vi "StarlyteWeatherLocationComparison.vi"() -> ()   [LabVIEW 2013]
doc: "# STARLYTE WEATHER LOCATION COMPARISON\n# SUBMITTED FOR 2017 NASA INTERNATIONAL SPACE APPS CHALLENGE\n# PROJECT: STARLYTE\n# AUTHORS: ANDREW DENIO\n# DATE: 5/5/2017"
uses:
  <vilib>/regexp/Match Regular Expression.xnode
panel:
  out "output string 3":string
  out "output string 2":string
  out "output string":string
  in  "stop":bool
  out "Fayetteville":picture
  out "HI-SEAs":picture
  out "element 126":string
  out "element 125":string
  out "element 124":string
  out "element 123":string
  out "element 122":string
  out "element 121":string
  out "element 120":string
  out "element 119":string
  out "element 118":string
  out "element 117":string
  out "element 116":string
  out "element 115":string
  out "element 114":string
  out "element 113":string
  out "element 112":string
  out "element 111":string
  out "element 110":string
  out "element 109":string
  out "element 84":string
  out "element 83":string
  out "element 82":string
  out "element 81":string
  out "element 80":string
  out "element 79":string
  out "element 78":string
  out "element 77":string
  out "element 76":string
  out "element 75":string
  out "element 74":string
  out "element 73":string
  out "element 72":string
  out "element 71":string
  out "element 70":string
  out "element 69":string
  out "element 68":string
  out "element 67":string
  out "element 66":string
  out "element 65":string
  out "element 64":string
  out "element 63":string
  out "element 62":string
  out "element 61":string
  out "element 60":string
  out "element 59":string
  out "element 58":string
  out "element 57":string
  out "element 56":string
  out "element 55":string
  out "element 54":string
  out "element 53":string
  out "element 52":string
  out "element 51":string
  out "element 50":string
  out "element 49":string
  out "element 48":string
  out "element 47":string
  out "element 46":string
  out "element 45":string
  out "element 44":string
  out "element 43":string
  out "element 42":string
  out "element 41":string
  out "element 40":string
  out "element 39":string
  out "element 38":string
  out "element 37":string
  out "element 36":string
  out "element 35":string
  out "element 34":string
  out "element 33":string
  out "element 32":string
  out "element 31":string
  out "element 30":string
  out "element 29":string
  out "element 28":string
  out "element 27":string
  out "element 26":string
  out "element 25":string
  out "element 24":string
  out "element 23":string
  out "element 22":string
  out "element 21":string
  out "element 20":string
  out "element 19":string
  out "element 18":string
  out "element 17":string
  out "element 16":string
  out "element 15":string
  out "element 14":string
  out "element 13":string
  out "element 12":string
  out "element 11":string
  out "element 10":string
  out "element 9":string
  out "element 8":string
  out "element 7":string
  out "element 6":string
  out "element 5":string
  out "element 4":string
  out "element 3":string
  out "element 2":string
  out "element":string
  # "HI-SEAs"
  # "Fayetteville"
  # "Space"
  # "Weather Location Comparison"
  # "Lattitude / Longitude:"
  # "Lattitude / Longitude:"
  # "Lattitude / Longitude:"
  # "Local Time:"
  # "Local Time:"
  # "Local Time:"
  # "Observation Time:"
  # "Observation Time:"
  # "Observation Time:"
  # "Station ID:"
  # "Station ID:"
  # "Station ID:"
  # "Local City:"
  # "Local City:"
  # "Local City:"
  # "Elevation:"
  # "Elevation:"
  # "Elevation:"
  # "Weather Alerts:"
  # "Weather Alerts:"
  # "Weather Alerts:"
  # "Condition:"
  # "Condition:"
  # "Condition:"
  # "Solar Radiation (W/m^2):"
  # "Solar Radiation (W/m^2):"
  # "Solar Radiation (W/m^2):"
  # "Current Temp (F):"
  # "Current Temp (F):"
  # "Current Temp (F):"
  # "Feels Like (F):"
  # "Feels Like (F):"
  # "Feels Like (F):"
  # "Wind Direction:"
  # "Wind Direction:"
  # "Wind Direction:"
  # "Wind Speed (mph):"
  # "Wind Speed (mph):"
  # "Wind Speed (mph):"
  # "Pressure (mb):"
  # "Pressure (mb):"
  # "Pressure (mb):"
  # "Precipitation (in):"
  # "Precipitation (in):"
  # "Precipitation (in):"
  # "Humidity:"
  # "Humidity:"
  # "Humidity:"
  # "Sunrise:"
  # "Sunrise:"
  # "Sunrise:"
  # "Sunset:"
  # "Sunset:"
  # "Sunset:"
  # "Instant Power:"
  # "Instant Power:"
  # "Instant Power:"
  # "Forecast:"
  # "Radar:"
  # "Forecast:"
  # "+1 Day:"
  # "+2 Days:"
  # "+3 Days:"
  # "+1 Day:"
  # "+2 Days:"
  # "+3 Days:"
  # "Condition:"
  # "Condition:"
  # "High Temp (F):"
  # "High Temp (F):"
  # "Low Temp (F):"
  # "Low Temp (F):"
  # "Chance of Rain (%):"
  # "Chance of Rain (%):"
  # "Rain level (in):"
  # "Rain level (in):"
  # "Wind Speed (mph):"
  # "Wind Speed (mph):"
  # "Wind Direction:"
  # "Wind Direction:"
  # "Avg Humidity (%)"
  # "Avg Humidity (%)"
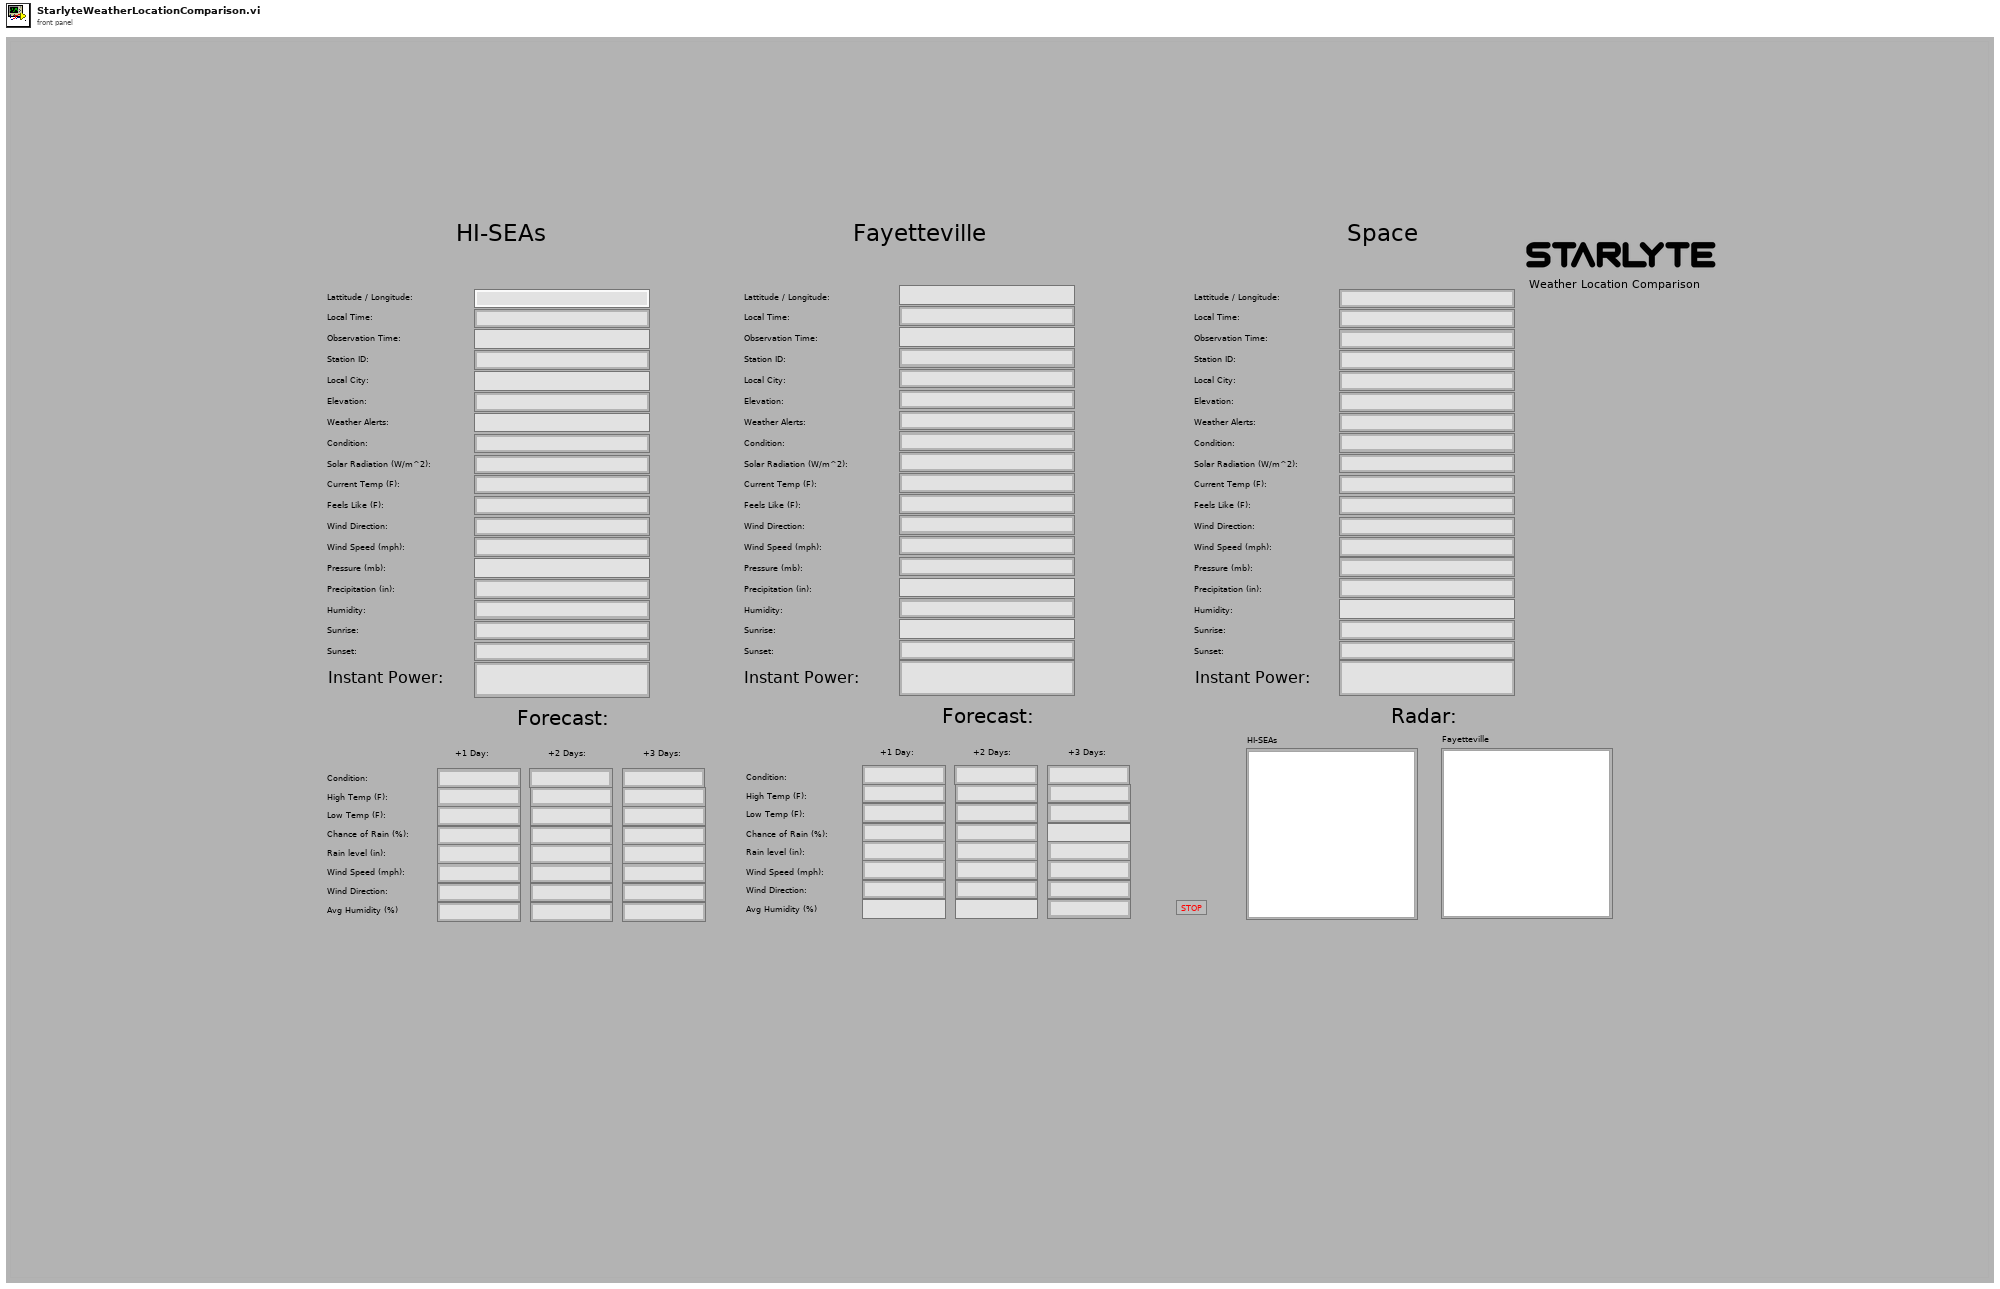
[diagram p1: front panel]
types:
  T1 = typedef "imagedata.ctl" = cluster{"image type":i32, "image depth":i32, "image":u8[], "mask":u8[], "colors":u32[], "Rectangle":cluster{"left":i16, "top":i16, "right":i16, "bottom":i16}}
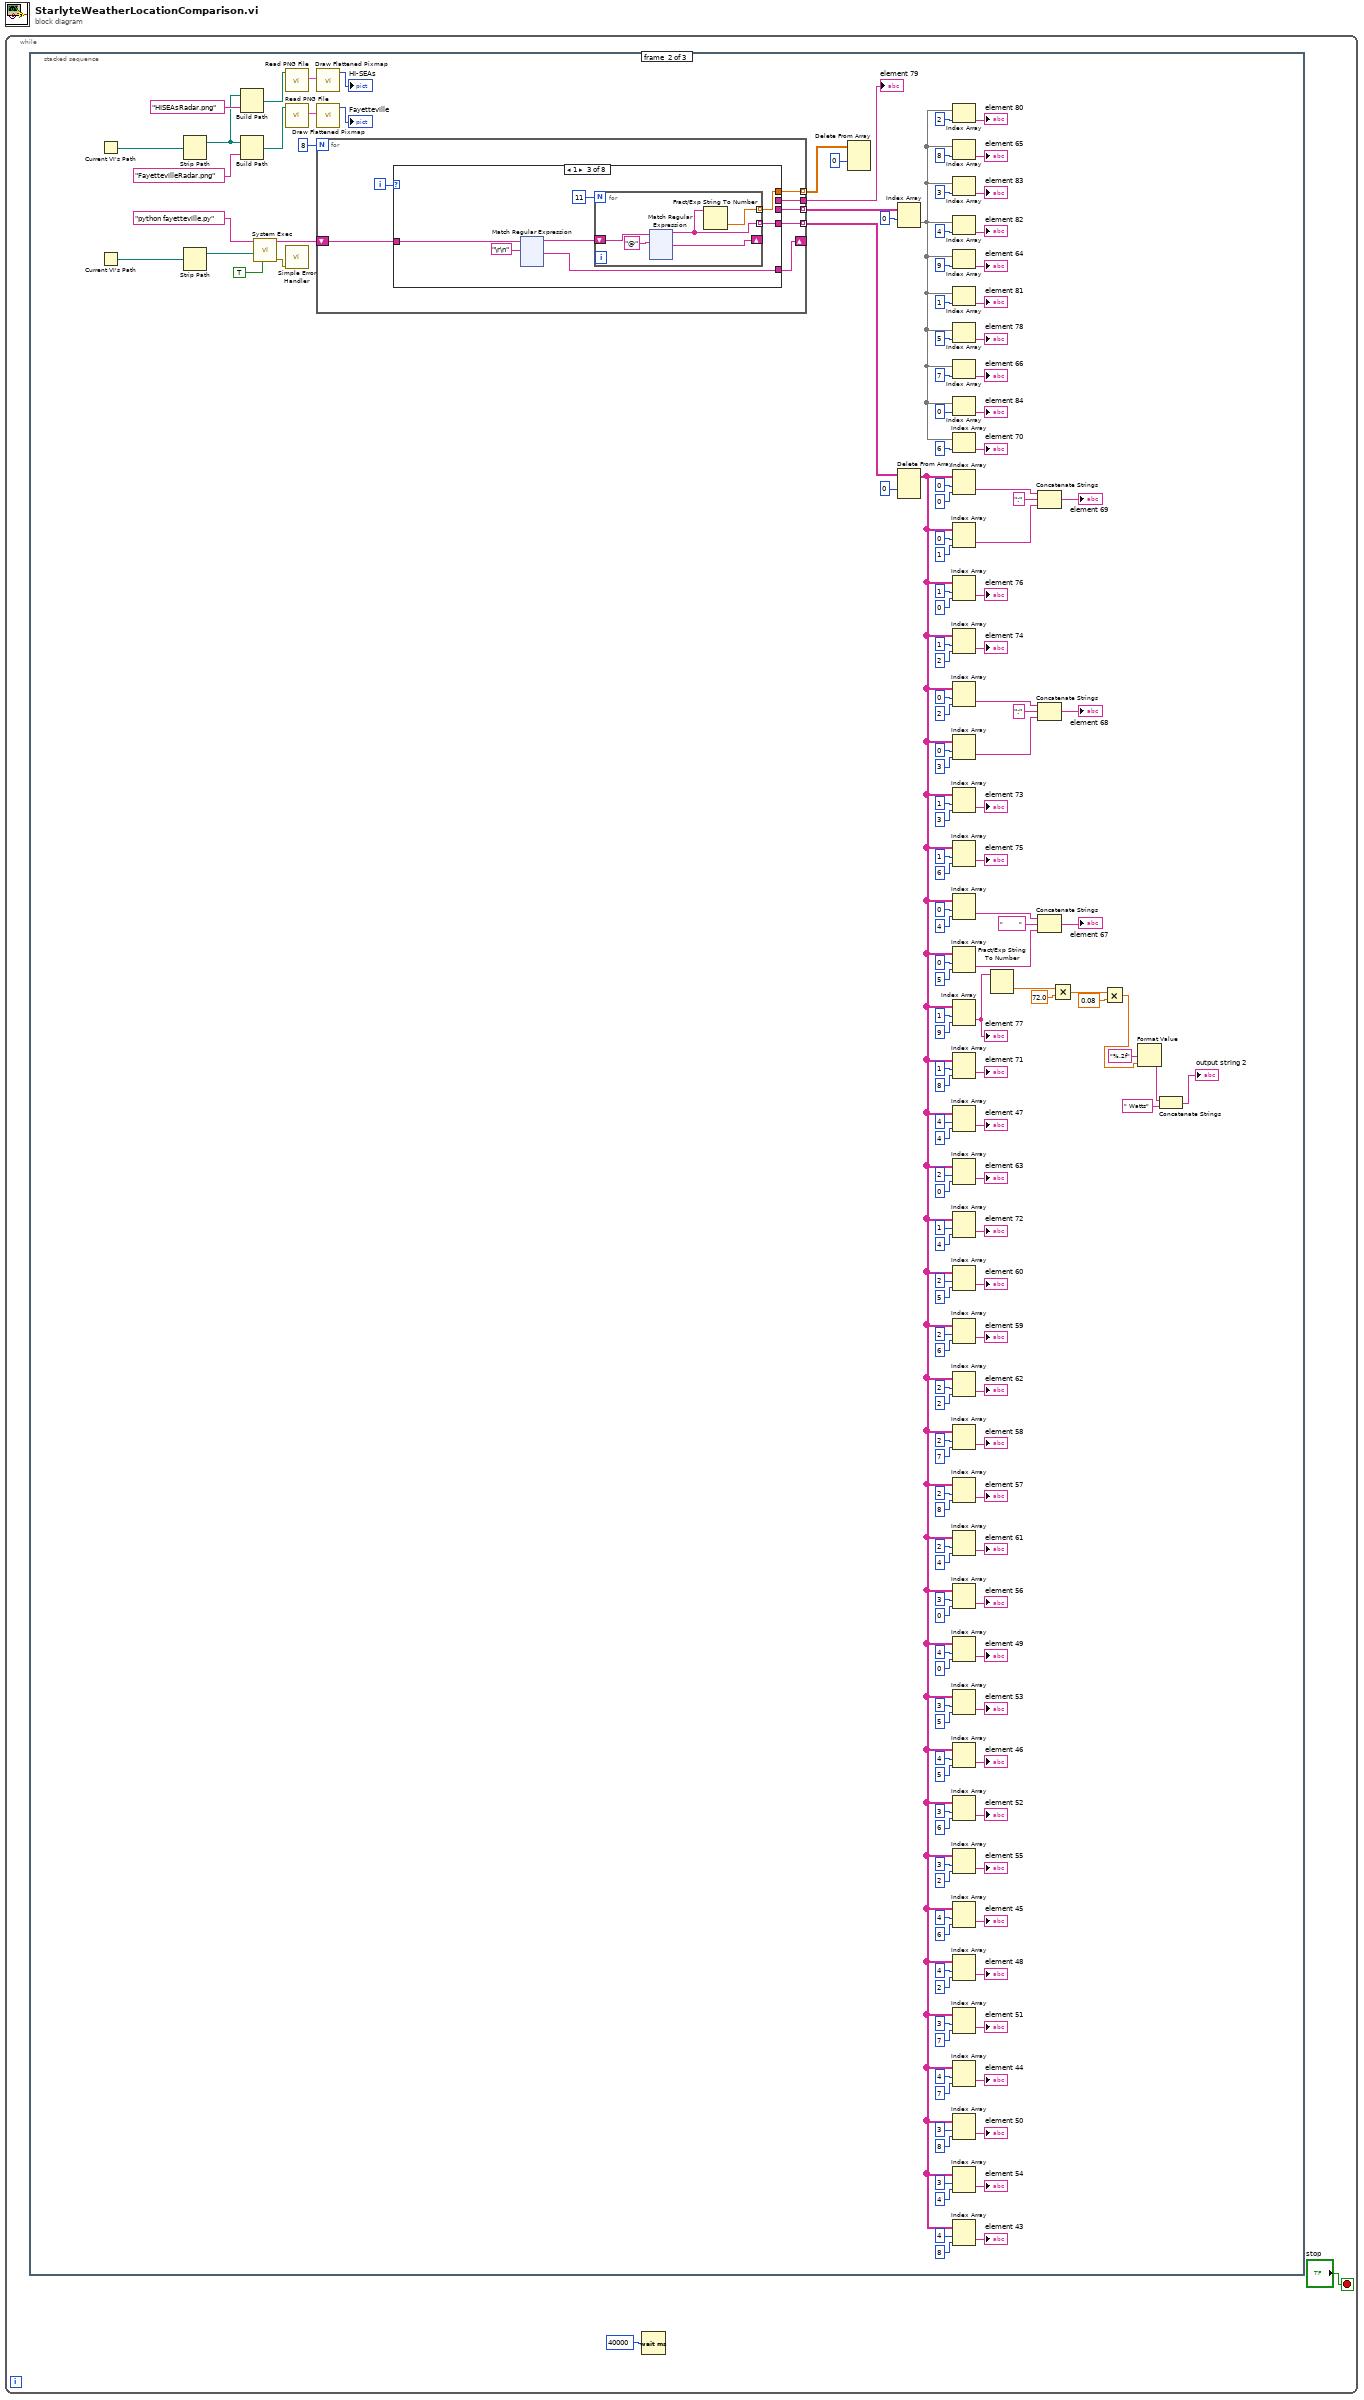
[diagram p0: block diagram]
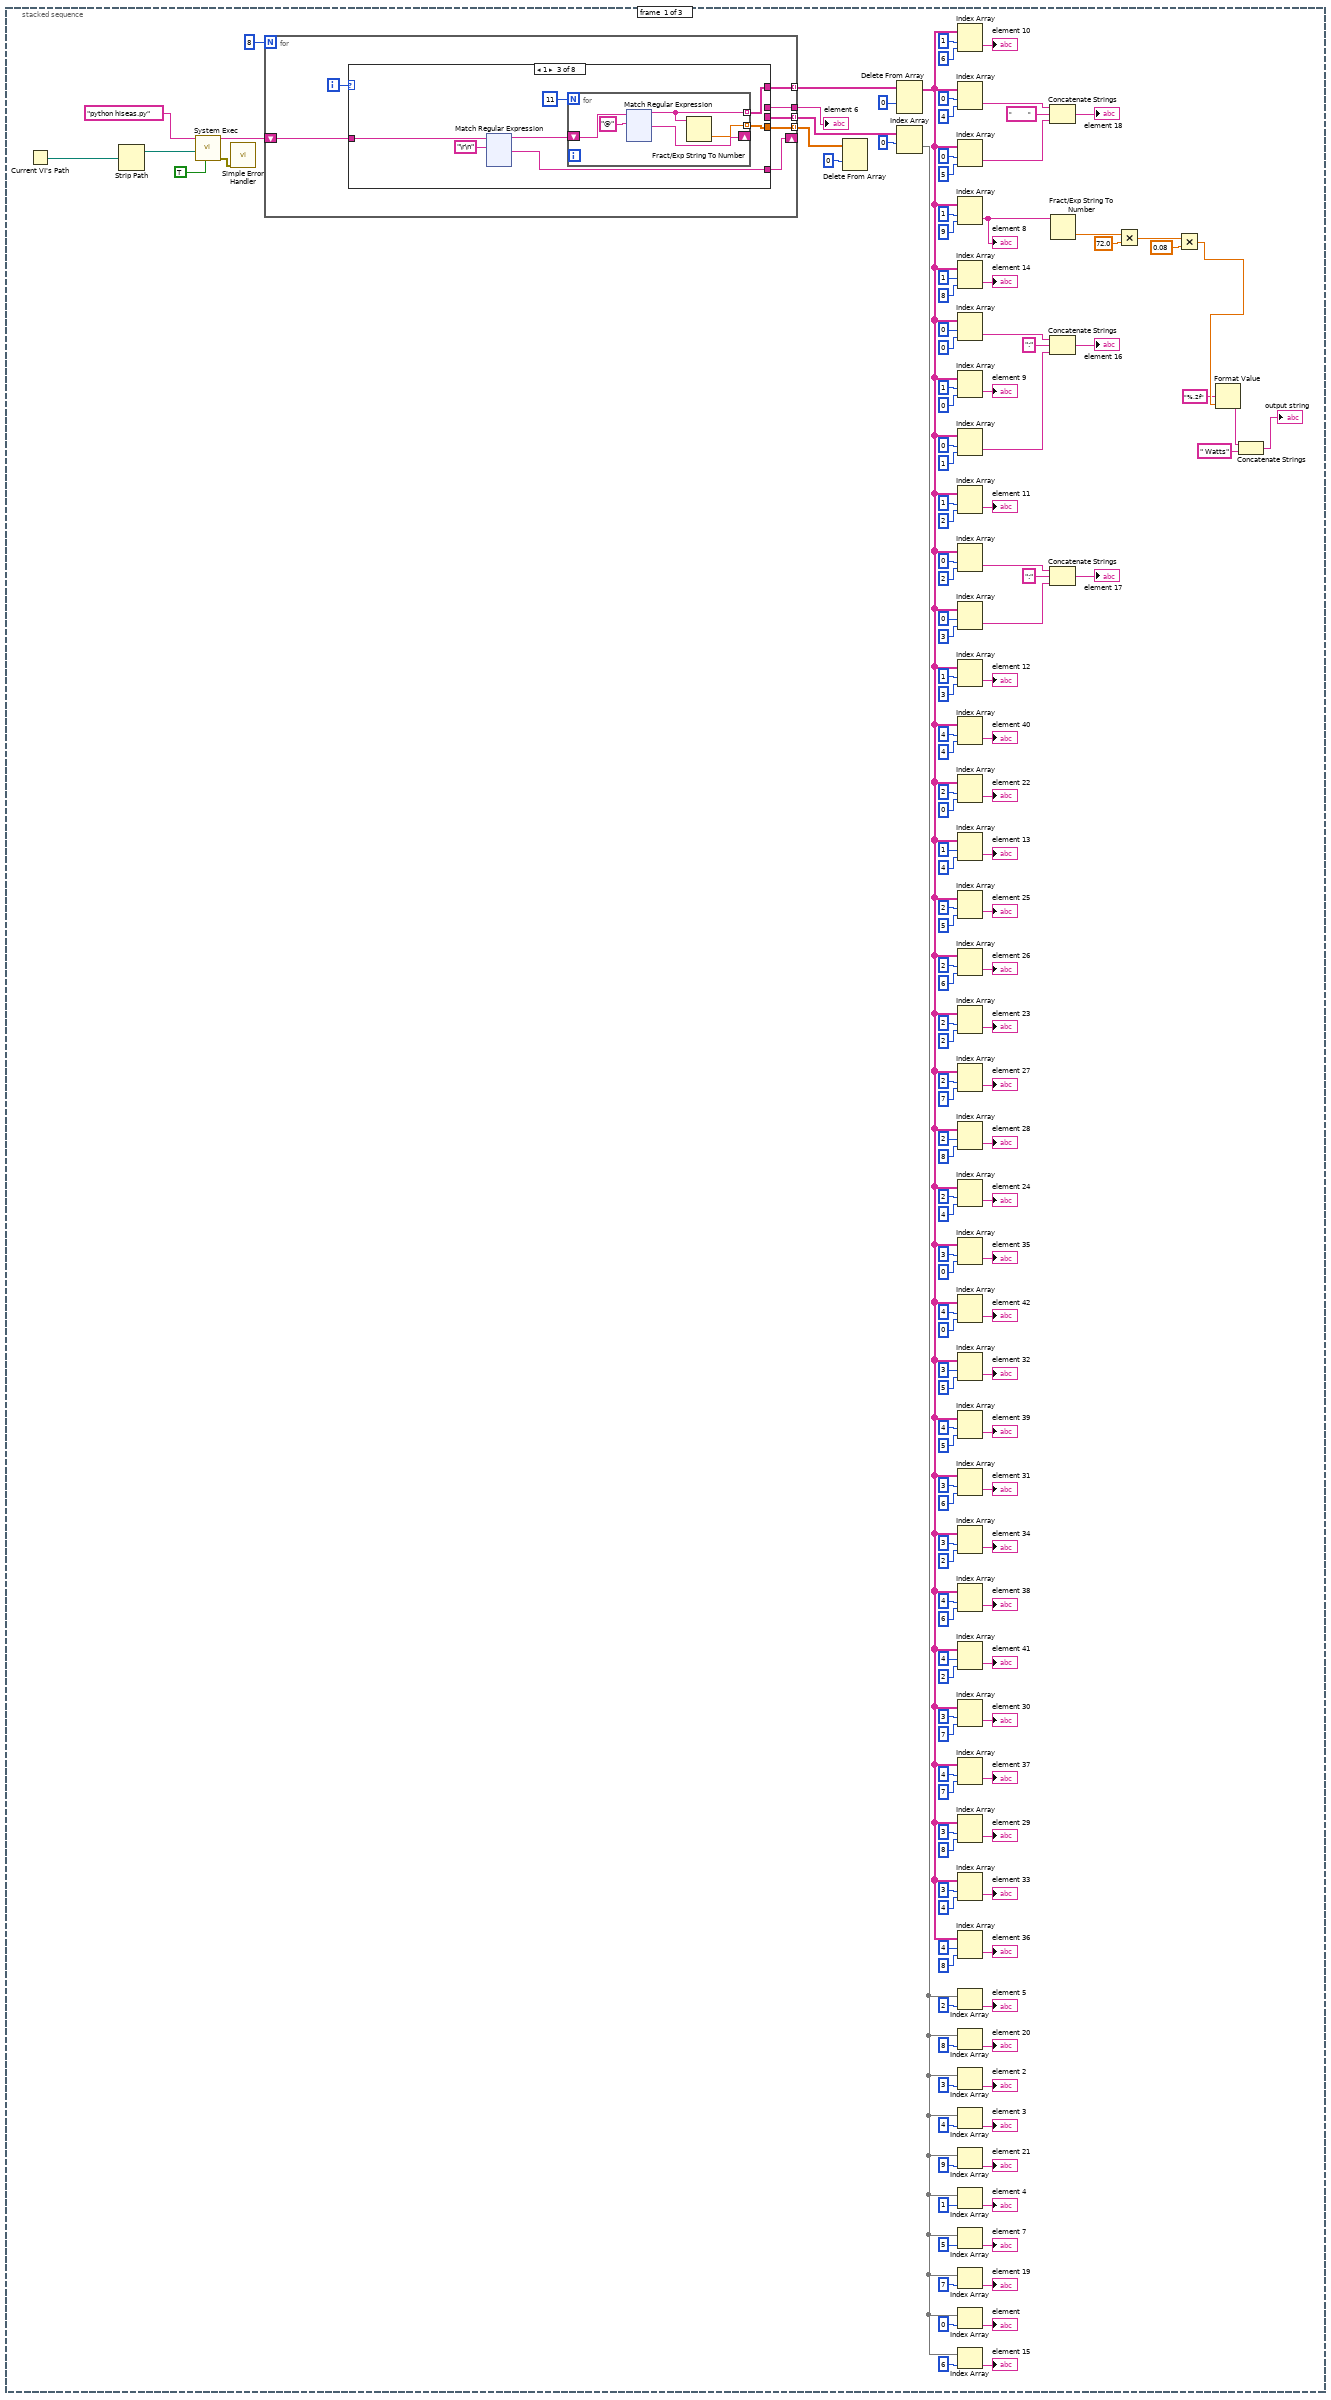
[diagram p2: hidden frame]
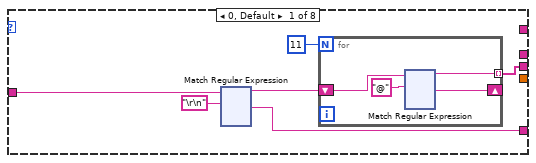
[diagram p3: hidden frame]
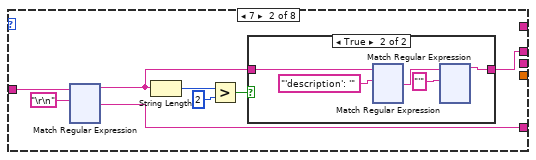
[diagram p4: hidden frame]
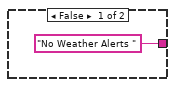
[diagram p5: hidden frame]
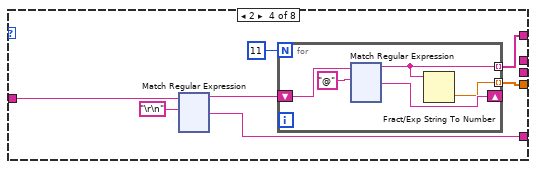
[diagram p6: hidden frame]
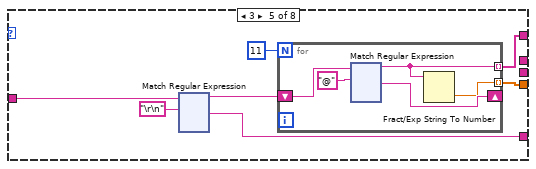
[diagram p7: hidden frame]
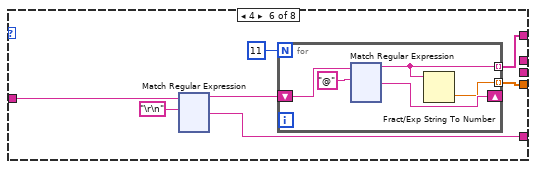
[diagram p8: hidden frame]
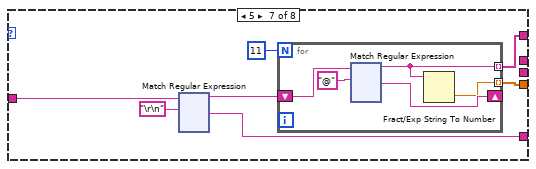
[diagram p9: hidden frame]
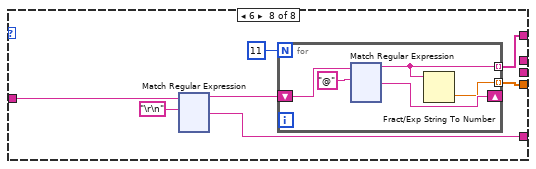
[diagram p10: hidden frame]
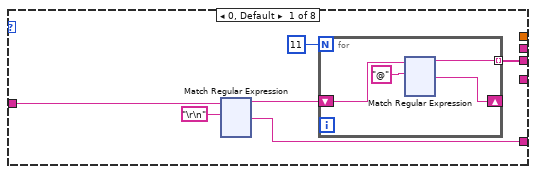
[diagram p11: hidden frame]
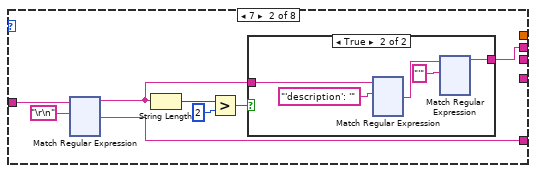
[diagram p12: hidden frame]
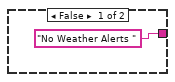
[diagram p13: hidden frame]
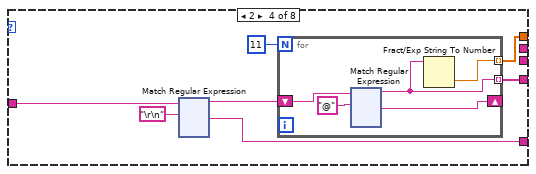
[diagram p14: hidden frame]
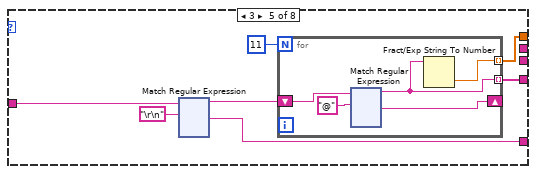
[diagram p15: hidden frame]
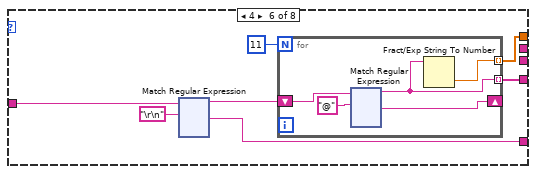
[diagram p16: hidden frame]
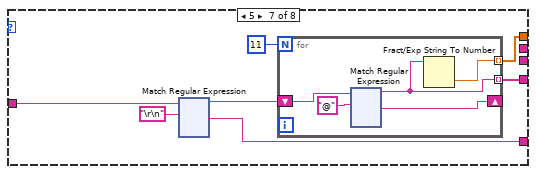
[diagram p17: hidden frame]
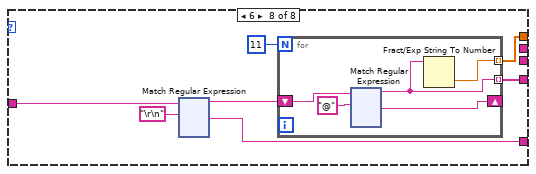
[diagram p18: hidden frame]
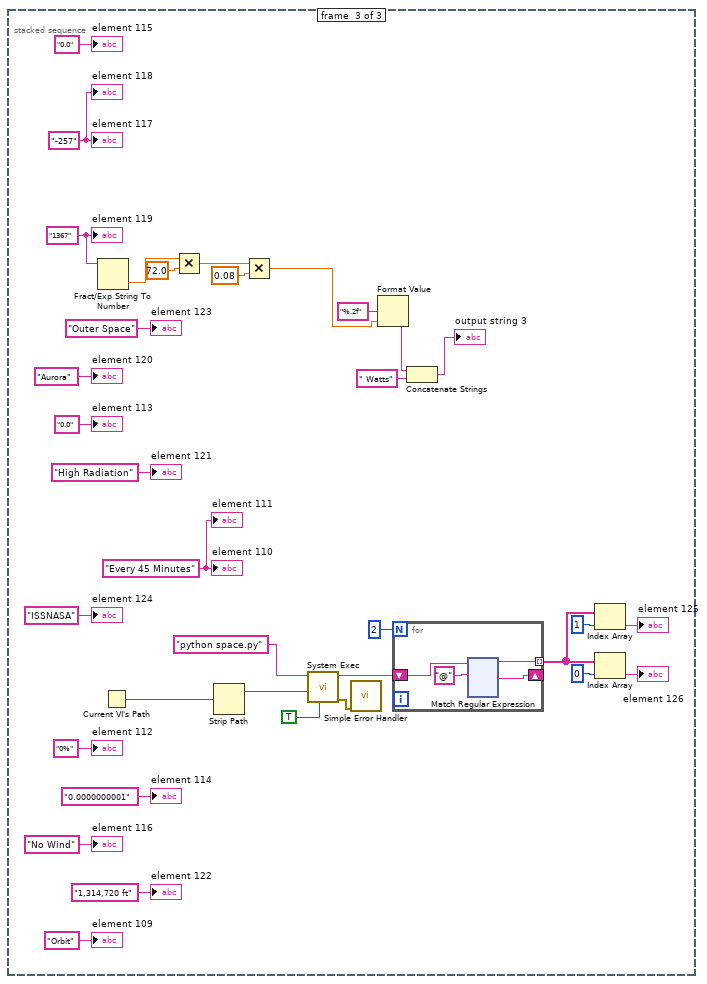
[diagram p19: hidden frame]
diagram:
  n1 = while {
    stop <- "stop" stop-if-true
    n2 = stacked-sequence {
      frame #0 {
        n3 = Current VI's Path() -> (path=w142:path)
        n4 = Strip Path(path=w142) -> (stripped path=w141:path)  [unwired: 1 out]
        n5 = call <vilib>:"System Exec.vi"("run minimized? (F)"=TRUE, "working directory"=w141, "command line"="python hiseas.py") -> ("error out"=w154:errorcluster, "standard output"=w152:string)  [unwired: 3 in, 4 out]
        n6 = call <vilib>:"Simple Error Handler.vi"("error in (no error)"=w154) -> ()  [unwired: 1 in, 8 out]
        n7 = for {
          N: 8 -> [_]
          shift-right: [w161] -> _
          shift-left: w152 -> [w162]
          tunnel: [w160] -> w149 mode=indexing
          tunnel: [w158] -> w148 mode=indexing
          tunnel: [w157] -> w133
          tunnel: [w156] -> w128 mode=indexing
          i -> [w159]
          n8 = case shown="1" w159 {
            tunnel: w162 -> [w167 w407 w762 w1002 w1242 w1482 w1722 w1962]
            tunnel: [w166 w406 w761 w1001 w1241 w1481 w1721 w1961] -> w161
            tunnel: [w164 _ _ _ _ _ _ _] -> w160
            tunnel: [_ _ w758 w998 w1238 w1478 w1718 w1958] -> w158
            tunnel: [_ w402 _ _ _ _ _ _] -> w157
            tunnel: [_ _ w757 w997 w1237 w1477 w1717 w1957] -> w156
            frame 0, Default {
              n9 = xnode "Match Regular Expression"("input string"=w167, "regular expression"="\r\n") -> ("before match"=w165:string, "after match"=w166:string)  [unwired: 4 in, 3 out]
              n10 = for {
                N: 11 -> [_]
                shift-right: [w170] -> _
                shift-left: w165 -> [w171]
                tunnel: [w169] -> w164 mode=indexing
                n11 = xnode "Match Regular Expression"("input string"=w171, "regular expression"="@") -> ("before match"=w169:string, "after match"=w170:string)  [unwired: 4 in, 3 out]
              }
            }
            frame 7 {
              n12 = xnode "Match Regular Expression"("input string"=w407, "regular expression"="\r\n") -> ("before match"=w401:string, "after match"=w406:string)  [unwired: 4 in, 3 out]
              n13 = String Length(string=w401) -> (length=w405:i32)
              n14 = Greater?(x=w405, y=2) -> (0:w403:bool)
              n15 = case shown="True" w403 {
                tunnel: ["No Weather Alerts " ("regular expression") w410] -> w402
                tunnel: w401 -> [_ w414]
                frame False {
                }
                frame True {
                  n16 = xnode "Match Regular Expression"("input string"=w414, "regular expression"="'description': '") -> ("after match"=w411:string)  [unwired: 4 in, 4 out]
                  n17 = xnode "Match Regular Expression"("input string"=w411, "regular expression"="'") -> ("before match"=w410:string)  [unwired: 4 in, 4 out]
                }
              }
            }
            frame 1 {
              n18 = xnode "Match Regular Expression"("input string"=w762, "regular expression"="\r\n") -> ("before match"=w760:string, "after match"=w761:string)  [unwired: 4 in, 3 out]
              n19 = for {
                N: 11 -> [_]
                shift-right: [w766] -> _
                shift-left: w760 -> [w767]
                tunnel: [w765] -> w758 mode=indexing
                tunnel: [w764] -> w757 mode=indexing
                n20 = xnode "Match Regular Expression"("input string"=w767, "regular expression"="@") -> ("before match"=w764:string, "after match"=w766:string)  [unwired: 4 in, 3 out]
                n21 = Fract/Exp String To Number(string=w764) -> (number=w765:dbl)  [unwired: 3 in, 1 out]
              }
            }
            frame 2 {
              n22 = xnode "Match Regular Expression"("input string"=w1002, "regular expression"="\r\n") -> ("before match"=w1000:string, "after match"=w1001:string)  [unwired: 4 in, 3 out]
              n23 = for {
                N: 11 -> [_]
                shift-right: [w1006] -> _
                shift-left: w1000 -> [w1007]
                tunnel: [w1005] -> w998 mode=indexing
                tunnel: [w1004] -> w997 mode=indexing
                n24 = xnode "Match Regular Expression"("input string"=w1007, "regular expression"="@") -> ("before match"=w1004:string, "after match"=w1006:string)  [unwired: 4 in, 3 out]
                n25 = Fract/Exp String To Number(string=w1004) -> (number=w1005:dbl)  [unwired: 3 in, 1 out]
              }
            }
            frame 3 {
              n26 = xnode "Match Regular Expression"("input string"=w1242, "regular expression"="\r\n") -> ("before match"=w1240:string, "after match"=w1241:string)  [unwired: 4 in, 3 out]
              n27 = for {
                N: 11 -> [_]
                shift-right: [w1246] -> _
                shift-left: w1240 -> [w1247]
                tunnel: [w1245] -> w1238 mode=indexing
                tunnel: [w1244] -> w1237 mode=indexing
                n28 = xnode "Match Regular Expression"("input string"=w1247, "regular expression"="@") -> ("before match"=w1244:string, "after match"=w1246:string)  [unwired: 4 in, 3 out]
                n29 = Fract/Exp String To Number(string=w1244) -> (number=w1245:dbl)  [unwired: 3 in, 1 out]
              }
            }
            frame 4 {
              n30 = xnode "Match Regular Expression"("input string"=w1482, "regular expression"="\r\n") -> ("before match"=w1480:string, "after match"=w1481:string)  [unwired: 4 in, 3 out]
              n31 = for {
                N: 11 -> [_]
                shift-right: [w1486] -> _
                shift-left: w1480 -> [w1487]
                tunnel: [w1485] -> w1478 mode=indexing
                tunnel: [w1484] -> w1477 mode=indexing
                n32 = xnode "Match Regular Expression"("input string"=w1487, "regular expression"="@") -> ("before match"=w1484:string, "after match"=w1486:string)  [unwired: 4 in, 3 out]
                n33 = Fract/Exp String To Number(string=w1484) -> (number=w1485:dbl)  [unwired: 3 in, 1 out]
              }
            }
            frame 5 {
              n34 = xnode "Match Regular Expression"("input string"=w1722, "regular expression"="\r\n") -> ("before match"=w1720:string, "after match"=w1721:string)  [unwired: 4 in, 3 out]
              n35 = for {
                N: 11 -> [_]
                shift-right: [w1726] -> _
                shift-left: w1720 -> [w1727]
                tunnel: [w1725] -> w1718 mode=indexing
                tunnel: [w1724] -> w1717 mode=indexing
                n36 = xnode "Match Regular Expression"("input string"=w1727, "regular expression"="@") -> ("before match"=w1724:string, "after match"=w1726:string)  [unwired: 4 in, 3 out]
                n37 = Fract/Exp String To Number(string=w1724) -> (number=w1725:dbl)  [unwired: 3 in, 1 out]
              }
            }
            frame 6 {
              n38 = xnode "Match Regular Expression"("input string"=w1962, "regular expression"="\r\n") -> ("before match"=w1960:string, "after match"=w1961:string)  [unwired: 4 in, 3 out]
              n39 = for {
                N: 11 -> [_]
                shift-right: [w1966] -> _
                shift-left: w1960 -> [w1967]
                tunnel: [w1965] -> w1958 mode=indexing
                tunnel: [w1964] -> w1957 mode=indexing
                n40 = xnode "Match Regular Expression"("input string"=w1967, "regular expression"="@") -> ("before match"=w1964:string, "after match"=w1966:string)  [unwired: 4 in, 3 out]
                n41 = Fract/Exp String To Number(string=w1964) -> (number=w1965:dbl)  [unwired: 3 in, 1 out]
              }
            }
          }
        }
        "element 6" <- w133
        n42 = Delete From Array(array=w148, index (row)=0) -> ()  [unwired: 2 in, 2 out]
        n43 = Delete From Array(array=w128, index (row)=0) -> (array with subset deleted=w14:string[][])  [unwired: 2 in, 1 out]
        n44 = Index Array(array=w149, index (row)=0 ("index")) -> (element=w13:string[])  [unwired: 1 in]
        n45 = Index Array(array=w14, index (row)=1, index (col)=6 ("disabled index (col)")) -> (element=→"element 10":string)
        n46 = Index Array(array=w14, index (row)=0, index (col)=4 ("disabled index (col)")) -> (element=w104:string)
        n47 = Index Array(array=w14, index (row)=0, index (col)=5 ("disabled index (col)")) -> (element=w106:string)
        n48 = Index Array(array=w14, index (row)=1, index (col)=9 ("disabled index (col)")) -> (element=w12:string)
        "element 8" <- w12
        n49 = Index Array(array=w14, index (row)=1, index (col)=8 ("disabled index (col)")) -> (element=→"element 14":string)
        n50 = Index Array(array=w14, index (row)=0, index (col)=0 ("disabled index (col)")) -> (element=w122:string)
        n51 = Index Array(array=w14, index (row)=1, index (col)=0 ("disabled index (col)")) -> (element=→"element 9":string)
        n52 = Index Array(array=w14, index (row)=0, index (col)=1 ("disabled index (col)")) -> (element=w121:string)
        n53 = Index Array(array=w14, index (row)=1, index (col)=2 ("disabled index (col)")) -> (element=→"element 11":string)
        n54 = Index Array(array=w14, index (row)=0, index (col)=2 ("disabled index (col)")) -> (element=w118:string)
        n55 = Index Array(array=w14, index (row)=0, index (col)=3 ("disabled index (col)")) -> (element=w119:string)
        n56 = Index Array(array=w14, index (row)=1, index (col)=3 ("disabled index (col)")) -> (element=→"element 12":string)
        n57 = Index Array(array=w14, index (row)=4, index (col)=4 ("disabled index (col)")) -> (element=→"element 40":string)
        n58 = Index Array(array=w14, index (row)=2, index (col)=0 ("disabled index (col)")) -> (element=→"element 22":string)
        n59 = Index Array(array=w14, index (row)=1, index (col)=4 ("disabled index (col)")) -> (element=→"element 13":string)
        n60 = Index Array(array=w14, index (row)=2, index (col)=5 ("disabled index (col)")) -> (element=→"element 25":string)
        n61 = Index Array(array=w14, index (row)=2, index (col)=6 ("disabled index (col)")) -> (element=→"element 26":string)
        n62 = Index Array(array=w14, index (row)=2, index (col)=2 ("disabled index (col)")) -> (element=→"element 23":string)
        n63 = Index Array(array=w14, index (row)=2, index (col)=7 ("disabled index (col)")) -> (element=→"element 27":string)
        n64 = Index Array(array=w14, index (row)=2, index (col)=8 ("disabled index (col)")) -> (element=→"element 28":string)
        n65 = Index Array(array=w14, index (row)=2, index (col)=4 ("disabled index (col)")) -> (element=→"element 24":string)
        n66 = Index Array(array=w14, index (row)=3, index (col)=0 ("disabled index (col)")) -> (element=→"element 35":string)
        n67 = Index Array(array=w14, index (row)=4, index (col)=0 ("disabled index (col)")) -> (element=→"element 42":string)
        n68 = Index Array(array=w14, index (row)=3, index (col)=5 ("disabled index (col)")) -> (element=→"element 32":string)
        n69 = Index Array(array=w14, index (row)=4, index (col)=5 ("disabled index (col)")) -> (element=→"element 39":string)
        n70 = Index Array(array=w14, index (row)=3, index (col)=6 ("disabled index (col)")) -> (element=→"element 31":string)
        n71 = Index Array(array=w14, index (row)=3, index (col)=2 ("disabled index (col)")) -> (element=→"element 34":string)
        n72 = Index Array(array=w14, index (row)=4, index (col)=6 ("disabled index (col)")) -> (element=→"element 38":string)
        n73 = Index Array(array=w14, index (row)=4, index (col)=2 ("disabled index (col)")) -> (element=→"element 41":string)
        n74 = Index Array(array=w14, index (row)=3, index (col)=7 ("disabled index (col)")) -> (element=→"element 30":string)
        n75 = Index Array(array=w14, index (row)=4, index (col)=7 ("disabled index (col)")) -> (element=→"element 37":string)
        n76 = Index Array(array=w14, index (row)=3, index (col)=8 ("disabled index (col)")) -> (element=→"element 29":string)
        n77 = Index Array(array=w14, index (row)=3, index (col)=4 ("disabled index (col)")) -> (element=→"element 33":string)
        n78 = Index Array(array=w14, index (row)=4, index (col)=8 ("disabled index (col)")) -> (element=→"element 36":string)
        n79 = Index Array(array=w13, index=2) -> (element=→"element 5":string)
        n80 = Index Array(array=w13, index=8 ("disabled index (col)")) -> (element=→"element 20":string)
        n81 = Index Array(array=w13, index=3) -> (element=→"element 2":string)
        n82 = Index Array(array=w13, index=4) -> (element=→"element 3":string)
        n83 = Index Array(array=w13, index=9 ("disabled index (col)")) -> (element=→"element 21":string)
        n84 = Index Array(array=w13, index=1) -> (element=→"element 4":string)
        n85 = Index Array(array=w13, index=5) -> (element=→"element 7":string)
        n86 = Index Array(array=w13, index=7 ("disabled index (col)")) -> (element=→"element 19":string)
        n87 = Index Array(array=w13, index=0) -> (element=→"element":string)
        n88 = Index Array(array=w13, index=6) -> (element=→"element 15":string)
        n89 = Concatenate Strings(w104, "        " ("string"), w106) -> (→"element 18":string)
        n90 = Concatenate Strings(w122, ":" ("string"), w121) -> (→"element 16":string)
        n91 = Concatenate Strings(w118, ":" ("string"), w119) -> (→"element 17":string)
        n92 = Fract/Exp String To Number(string=w12) -> (number=w11:dbl)  [unwired: 3 in, 1 out]
        n93 = Multiply(x=w11, y=72.0) -> (x*y=w9:dbl)
        n94 = Multiply(x=w9, y=0.08) -> (x*y=w7:dbl)
        n95 = Format Value(format string="%.2f", value (0)=w7) -> (output string=w6:string)  [unwired: 1 in]
        n96 = Concatenate Strings(w6, " Watts" ("string")) -> (→"output string":string)
      }
      frame #1 {
        n97 = Current VI's Path() -> (path=w2216:path)
        n98 = Current VI's Path() -> (path=w2346:path)
        n99 = Strip Path(path=w2216) -> (stripped path=w2209:path)  [unwired: 1 out]
        n100 = Strip Path(path=w2346) -> (stripped path=w2345:path)  [unwired: 1 out]
        n101 = Build Path(base path=w2209, name or relative path="HISEAsRadar.png") -> (appended path=w2208:path)
        n102 = Build Path(base path=w2209, name or relative path="FayettevilleRadar.png") -> (appended path=w2211:path)
        n103 = call <vilib>:"System Exec.vi"("run minimized? (F)"=TRUE, "working directory"=w2345, "command line"="python fayetteville.py") -> ("error out"=w2358:errorcluster, "standard output"=w2356:string)  [unwired: 3 in, 4 out]
        n104 = call <vilib>:"Read PNG File.vi"("path to PNG file"=w2208) -> ("image data"=w2213:T1)  [unwired: 8 in, 2 out]
        n105 = call <vilib>:"Read PNG File.vi"("path to PNG file"=w2211) -> ("image data"=w2212:T1)  [unwired: 8 in, 2 out]
        n106 = call <vilib>:"Simple Error Handler.vi"("error in (no error)"=w2358) -> ()  [unwired: 1 in, 8 out]
        n107 = call <vilib>:"Draw Flattened Pixmap.vi"("image data"=w2213) -> ("new picture"=→"HI-SEAs":picture)  [unwired: 8 in]
        n108 = call <vilib>:"Draw Flattened Pixmap.vi"("image data"=w2212) -> ("new picture"=→"Fayetteville":picture)  [unwired: 8 in]
        n109 = for {
          N: 8 -> [_]
          shift-right: [w2365] -> _
          shift-left: w2356 -> [w2366]
          tunnel: [w2364] -> w2353 mode=indexing
          tunnel: [w2362] -> w2352 mode=indexing
          tunnel: [w2361] -> w2337
          tunnel: [w2360] -> w2332 mode=indexing
          i -> [w2363]
          n110 = case shown="1" w2363 {
            tunnel: w2366 -> [w2371 w2611 w2966 w3206 w3446 w3686 w3926 w4166]
            tunnel: [w2370 w2610 w2965 w3205 w3445 w3685 w3925 w4165] -> w2365
            tunnel: [w2368 _ _ _ _ _ _ _] -> w2364
            tunnel: [_ _ w2962 w3202 w3442 w3682 w3922 w4162] -> w2362
            tunnel: [_ w2606 _ _ _ _ _ _] -> w2361
            tunnel: [_ _ w2961 w3201 w3441 w3681 w3921 w4161] -> w2360
            frame 0, Default {
              n111 = xnode "Match Regular Expression"("input string"=w2371, "regular expression"="\r\n") -> ("before match"=w2369:string, "after match"=w2370:string)  [unwired: 4 in, 3 out]
              n112 = for {
                N: 11 -> [_]
                shift-right: [w2374] -> _
                shift-left: w2369 -> [w2375]
                tunnel: [w2373] -> w2368 mode=indexing
                n113 = xnode "Match Regular Expression"("input string"=w2375, "regular expression"="@") -> ("before match"=w2373:string, "after match"=w2374:string)  [unwired: 4 in, 3 out]
              }
            }
            frame 7 {
              n114 = xnode "Match Regular Expression"("input string"=w2611, "regular expression"="\r\n") -> ("before match"=w2605:string, "after match"=w2610:string)  [unwired: 4 in, 3 out]
              n115 = String Length(string=w2605) -> (length=w2609:i32)
              n116 = Greater?(x=w2609, y=2) -> (0:w2607:bool)
              n117 = case shown="True" w2607 {
                tunnel: ["No Weather Alerts " ("regular expression") w2614] -> w2606
                tunnel: w2605 -> [_ w2618]
                frame False {
                }
                frame True {
                  n118 = xnode "Match Regular Expression"("input string"=w2618, "regular expression"="'description': '") -> ("after match"=w2615:string)  [unwired: 4 in, 4 out]
                  n119 = xnode "Match Regular Expression"("input string"=w2615, "regular expression"="'") -> ("before match"=w2614:string)  [unwired: 4 in, 4 out]
                }
              }
            }
            frame 1 {
              n120 = xnode "Match Regular Expression"("input string"=w2966, "regular expression"="\r\n") -> ("before match"=w2964:string, "after match"=w2965:string)  [unwired: 4 in, 3 out]
              n121 = for {
                N: 11 -> [_]
                shift-right: [w2970] -> _
                shift-left: w2964 -> [w2971]
                tunnel: [w2969] -> w2962 mode=indexing
                tunnel: [w2968] -> w2961 mode=indexing
                n122 = xnode "Match Regular Expression"("input string"=w2971, "regular expression"="@") -> ("before match"=w2968:string, "after match"=w2970:string)  [unwired: 4 in, 3 out]
                n123 = Fract/Exp String To Number(string=w2968) -> (number=w2969:dbl)  [unwired: 3 in, 1 out]
              }
            }
            frame 2 {
              n124 = xnode "Match Regular Expression"("input string"=w3206, "regular expression"="\r\n") -> ("before match"=w3204:string, "after match"=w3205:string)  [unwired: 4 in, 3 out]
              n125 = for {
                N: 11 -> [_]
                shift-right: [w3210] -> _
                shift-left: w3204 -> [w3211]
                tunnel: [w3209] -> w3202 mode=indexing
                tunnel: [w3208] -> w3201 mode=indexing
                n126 = xnode "Match Regular Expression"("input string"=w3211, "regular expression"="@") -> ("before match"=w3208:string, "after match"=w3210:string)  [unwired: 4 in, 3 out]
                n127 = Fract/Exp String To Number(string=w3208) -> (number=w3209:dbl)  [unwired: 3 in, 1 out]
              }
            }
            frame 3 {
              n128 = xnode "Match Regular Expression"("input string"=w3446, "regular expression"="\r\n") -> ("before match"=w3444:string, "after match"=w3445:string)  [unwired: 4 in, 3 out]
              n129 = for {
                N: 11 -> [_]
                shift-right: [w3450] -> _
                shift-left: w3444 -> [w3451]
                tunnel: [w3449] -> w3442 mode=indexing
                tunnel: [w3448] -> w3441 mode=indexing
                n130 = xnode "Match Regular Expression"("input string"=w3451, "regular expression"="@") -> ("before match"=w3448:string, "after match"=w3450:string)  [unwired: 4 in, 3 out]
                n131 = Fract/Exp String To Number(string=w3448) -> (number=w3449:dbl)  [unwired: 3 in, 1 out]
              }
            }
            frame 4 {
              n132 = xnode "Match Regular Expression"("input string"=w3686, "regular expression"="\r\n") -> ("before match"=w3684:string, "after match"=w3685:string)  [unwired: 4 in, 3 out]
              n133 = for {
                N: 11 -> [_]
                shift-right: [w3690] -> _
                shift-left: w3684 -> [w3691]
                tunnel: [w3689] -> w3682 mode=indexing
                tunnel: [w3688] -> w3681 mode=indexing
                n134 = xnode "Match Regular Expression"("input string"=w3691, "regular expression"="@") -> ("before match"=w3688:string, "after match"=w3690:string)  [unwired: 4 in, 3 out]
                n135 = Fract/Exp String To Number(string=w3688) -> (number=w3689:dbl)  [unwired: 3 in, 1 out]
              }
            }
            frame 5 {
              n136 = xnode "Match Regular Expression"("input string"=w3926, "regular expression"="\r\n") -> ("before match"=w3924:string, "after match"=w3925:string)  [unwired: 4 in, 3 out]
              n137 = for {
                N: 11 -> [_]
                shift-right: [w3930] -> _
                shift-left: w3924 -> [w3931]
                tunnel: [w3929] -> w3922 mode=indexing
                tunnel: [w3928] -> w3921 mode=indexing
                n138 = xnode "Match Regular Expression"("input string"=w3931, "regular expression"="@") -> ("before match"=w3928:string, "after match"=w3930:string)  [unwired: 4 in, 3 out]
                n139 = Fract/Exp String To Number(string=w3928) -> (number=w3929:dbl)  [unwired: 3 in, 1 out]
              }
            }
            frame 6 {
              n140 = xnode "Match Regular Expression"("input string"=w4166, "regular expression"="\r\n") -> ("before match"=w4164:string, "after match"=w4165:string)  [unwired: 4 in, 3 out]
              n141 = for {
                N: 11 -> [_]
                shift-right: [w4170] -> _
                shift-left: w4164 -> [w4171]
                tunnel: [w4169] -> w4162 mode=indexing
                tunnel: [w4168] -> w4161 mode=indexing
                n142 = xnode "Match Regular Expression"("input string"=w4171, "regular expression"="@") -> ("before match"=w4168:string, "after match"=w4170:string)  [unwired: 4 in, 3 out]
                n143 = Fract/Exp String To Number(string=w4168) -> (number=w4169:dbl)  [unwired: 3 in, 1 out]
              }
            }
          }
        }
        "element 79" <- w2337
        n144 = Delete From Array(array=w2352, index (row)=0) -> ()  [unwired: 2 in, 2 out]
        n145 = Index Array(array=w2353, index (row)=0 ("index")) -> (element=w2217:string[])  [unwired: 1 in]
        n146 = Delete From Array(array=w2332, index (row)=0) -> (array with subset deleted=w2218:string[][])  [unwired: 2 in, 1 out]
        n147 = Index Array(array=w2217, index=2) -> (element=→"element 80":string)
        n148 = Index Array(array=w2217, index=8 ("disabled index (col)")) -> (element=→"element 65":string)
        n149 = Index Array(array=w2217, index=3) -> (element=→"element 83":string)
        n150 = Index Array(array=w2217, index=4) -> (element=→"element 82":string)
        n151 = Index Array(array=w2217, index=9 ("disabled index (col)")) -> (element=→"element 64":string)
        n152 = Index Array(array=w2217, index=1) -> (element=→"element 81":string)
        n153 = Index Array(array=w2217, index=5) -> (element=→"element 78":string)
        n154 = Index Array(array=w2217, index=7 ("disabled index (col)")) -> (element=→"element 66":string)
        n155 = Index Array(array=w2217, index=0) -> (element=→"element 84":string)
        n156 = Index Array(array=w2217, index=6) -> (element=→"element 70":string)
        n157 = Index Array(array=w2218, index (row)=0, index (col)=0 ("disabled index (col)")) -> (element=w2326:string)
        n158 = Index Array(array=w2218, index (row)=0, index (col)=1 ("disabled index (col)")) -> (element=w2325:string)
        n159 = Index Array(array=w2218, index (row)=1, index (col)=0 ("disabled index (col)")) -> (element=→"element 76":string)
        n160 = Index Array(array=w2218, index (row)=1, index (col)=2 ("disabled index (col)")) -> (element=→"element 74":string)
        n161 = Index Array(array=w2218, index (row)=0, index (col)=2 ("disabled index (col)")) -> (element=w2322:string)
        n162 = Index Array(array=w2218, index (row)=0, index (col)=3 ("disabled index (col)")) -> (element=w2323:string)
        n163 = Index Array(array=w2218, index (row)=1, index (col)=3 ("disabled index (col)")) -> (element=→"element 73":string)
        n164 = Index Array(array=w2218, index (row)=1, index (col)=6 ("disabled index (col)")) -> (element=→"element 75":string)
        n165 = Index Array(array=w2218, index (row)=0, index (col)=4 ("disabled index (col)")) -> (element=w2308:string)
        n166 = Index Array(array=w2218, index (row)=0, index (col)=5 ("disabled index (col)")) -> (element=w2310:string)
        n167 = Index Array(array=w2218, index (row)=1, index (col)=9 ("disabled index (col)")) -> (element=w2202:string)
        "element 77" <- w2202
        n168 = Index Array(array=w2218, index (row)=1, index (col)=8 ("disabled index (col)")) -> (element=→"element 71":string)
        n169 = Index Array(array=w2218, index (row)=4, index (col)=4 ("disabled index (col)")) -> (element=→"element 47":string)
        n170 = Index Array(array=w2218, index (row)=2, index (col)=0 ("disabled index (col)")) -> (element=→"element 63":string)
        n171 = Index Array(array=w2218, index (row)=1, index (col)=4 ("disabled index (col)")) -> (element=→"element 72":string)
        n172 = Index Array(array=w2218, index (row)=2, index (col)=5 ("disabled index (col)")) -> (element=→"element 60":string)
        n173 = Index Array(array=w2218, index (row)=2, index (col)=6 ("disabled index (col)")) -> (element=→"element 59":string)
        n174 = Index Array(array=w2218, index (row)=2, index (col)=2 ("disabled index (col)")) -> (element=→"element 62":string)
        n175 = Index Array(array=w2218, index (row)=2, index (col)=7 ("disabled index (col)")) -> (element=→"element 58":string)
        n176 = Index Array(array=w2218, index (row)=2, index (col)=8 ("disabled index (col)")) -> (element=→"element 57":string)
        n177 = Index Array(array=w2218, index (row)=2, index (col)=4 ("disabled index (col)")) -> (element=→"element 61":string)
        n178 = Index Array(array=w2218, index (row)=3, index (col)=0 ("disabled index (col)")) -> (element=→"element 56":string)
        n179 = Index Array(array=w2218, index (row)=4, index (col)=0 ("disabled index (col)")) -> (element=→"element 49":string)
        n180 = Index Array(array=w2218, index (row)=3, index (col)=5 ("disabled index (col)")) -> (element=→"element 53":string)
        n181 = Index Array(array=w2218, index (row)=4, index (col)=5 ("disabled index (col)")) -> (element=→"element 46":string)
        n182 = Index Array(array=w2218, index (row)=3, index (col)=6 ("disabled index (col)")) -> (element=→"element 52":string)
        n183 = Index Array(array=w2218, index (row)=3, index (col)=2 ("disabled index (col)")) -> (element=→"element 55":string)
        n184 = Index Array(array=w2218, index (row)=4, index (col)=6 ("disabled index (col)")) -> (element=→"element 45":string)
        n185 = Index Array(array=w2218, index (row)=4, index (col)=2 ("disabled index (col)")) -> (element=→"element 48":string)
        n186 = Index Array(array=w2218, index (row)=3, index (col)=7 ("disabled index (col)")) -> (element=→"element 51":string)
        n187 = Index Array(array=w2218, index (row)=4, index (col)=7 ("disabled index (col)")) -> (element=→"element 44":string)
        n188 = Index Array(array=w2218, index (row)=3, index (col)=8 ("disabled index (col)")) -> (element=→"element 50":string)
        n189 = Index Array(array=w2218, index (row)=3, index (col)=4 ("disabled index (col)")) -> (element=→"element 54":string)
        n190 = Index Array(array=w2218, index (row)=4, index (col)=8 ("disabled index (col)")) -> (element=→"element 43":string)
        n191 = Fract/Exp String To Number(string=w2202) -> (number=w2203:dbl)  [unwired: 3 in, 1 out]
        n192 = Concatenate Strings(w2326, ":" ("string"), w2325) -> (→"element 69":string)
        n193 = Concatenate Strings(w2322, ":" ("string"), w2323) -> (→"element 68":string)
        n194 = Concatenate Strings(w2308, "        " ("string"), w2310) -> (→"element 67":string)
        n195 = Multiply(x=w2203, y=72.0) -> (x*y=w2205:dbl)
        n196 = Multiply(x=w2205, y=0.08) -> (x*y=w2197:dbl)
        n197 = Format Value(format string="%.2f", value (0)=w2197) -> (output string=w2198:string)  [unwired: 1 in]
        n198 = Concatenate Strings(w2198, " Watts" ("string")) -> (→"output string 2":string)
      }
      frame #2 {
        w4417 = "Every 45 Minutes" ("element 111")
        w4423 = "-257" ("element 118")
        w4406 = "1367" ("element 119")
        n199 = Fract/Exp String To Number(string=w4406) -> (number=w4407:dbl)  [unwired: 3 in, 1 out]
        n200 = Current VI's Path() -> (path=w4430:path)
        n201 = Multiply(x=w4407, y=72.0) -> (x*y=w4409:dbl)
        n202 = Strip Path(path=w4430) -> (stripped path=w4429:path)  [unwired: 1 out]
        n203 = Multiply(x=w4409, y=0.08) -> (x*y=w4401:dbl)
        n204 = call <vilib>:"System Exec.vi"("run minimized? (F)"=TRUE, "working directory"=w4429, "command line"="python space.py") -> ("error out"=w4434:errorcluster, "standard output"=w4414:string)  [unwired: 3 in, 4 out]
        n205 = call <vilib>:"Simple Error Handler.vi"("error in (no error)"=w4434) -> ()  [unwired: 1 in, 8 out]
        n206 = Format Value(format string="%.2f", value (0)=w4401) -> (output string=w4402:string)  [unwired: 1 in]
        n207 = for {
          N: 2 -> [_]
          shift-right: [w4437] -> _
          shift-left: w4414 -> [w4438]
          tunnel: [w4436] -> w4413 mode=indexing
          n208 = xnode "Match Regular Expression"("input string"=w4438, "regular expression"="@") -> ("before match"=w4436:string, "after match"=w4437:string)  [unwired: 4 in, 3 out]
        }
        n209 = Concatenate Strings(w4402, " Watts" ("string")) -> (→"output string 3":string)
        n210 = Index Array(array=w4413, index=1) -> (element=→"element 125":string)
        n211 = Index Array(array=w4413, index=0) -> (element=→"element 126":string)
        "element 124" <- "ISSNASA" ("element 124")
        "element 123" <- "Outer Space" ("element 123")
        "element 122" <- "1,314,720 ft" ("element 122")
        "element 121" <- "High Radiation" ("element 121")
        "element 120" <- "Aurora" ("element 120")
        "element 119" <- w4406
        "element 118" <- w4423
        "element 117" <- w4423
        "element 116" <- "No Wind" ("element 116")
        "element 115" <- "0.0" ("element 115")
        "element 114" <- "0.0000000001" ("element 114")
        "element 113" <- "0.0" ("element 113")
        "element 112" <- "0%" ("element 112")
        "element 111" <- w4417
        "element 110" <- w4417
        "element 109" <- "Orbit" ("string")
      }
    }
    n212 = Wait (ms)(milliseconds to wait=u32 40000) -> ()  [unwired: 1 out]
  }
